vi "TLB Native Dynamic Events ver 0.26d.vi"() -> ()   [LabVIEW 2018] (continued)
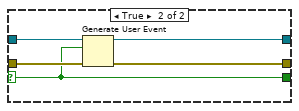
[diagram p2: hidden frame]
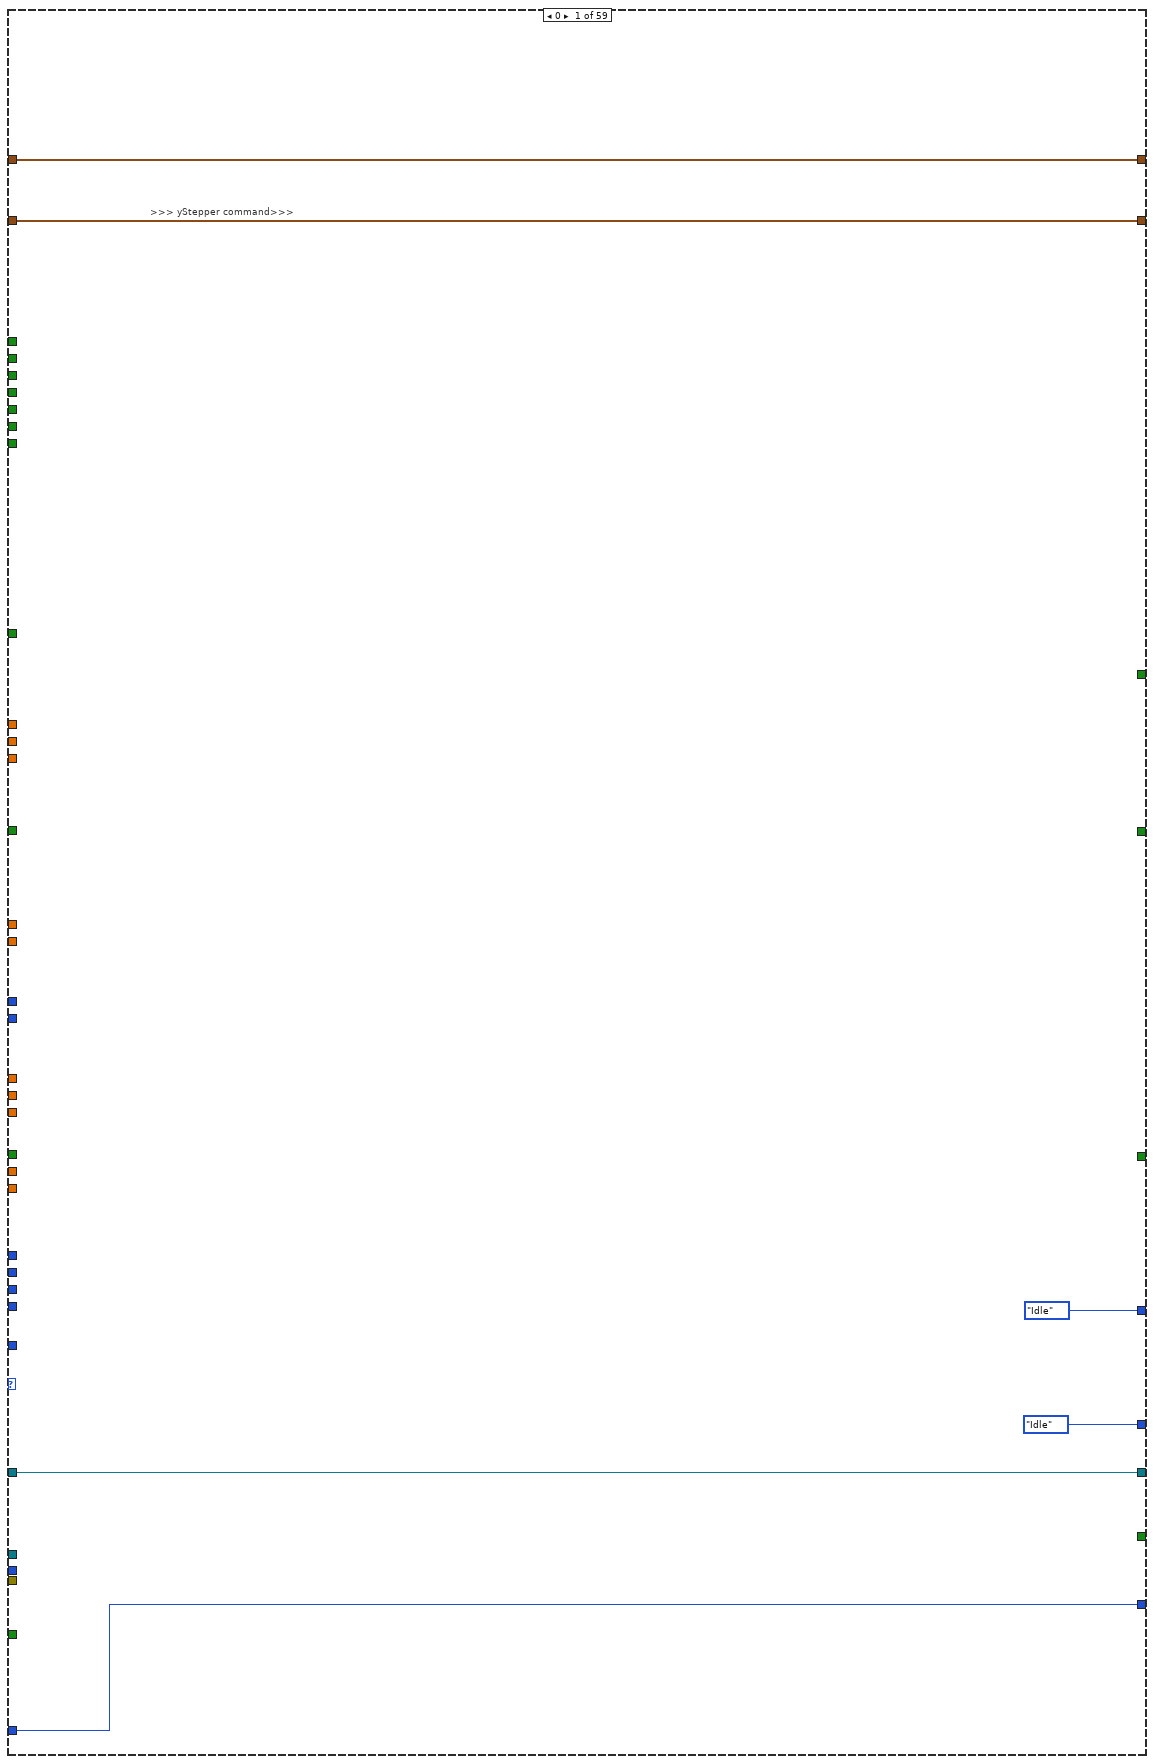
[diagram p5: hidden frame]
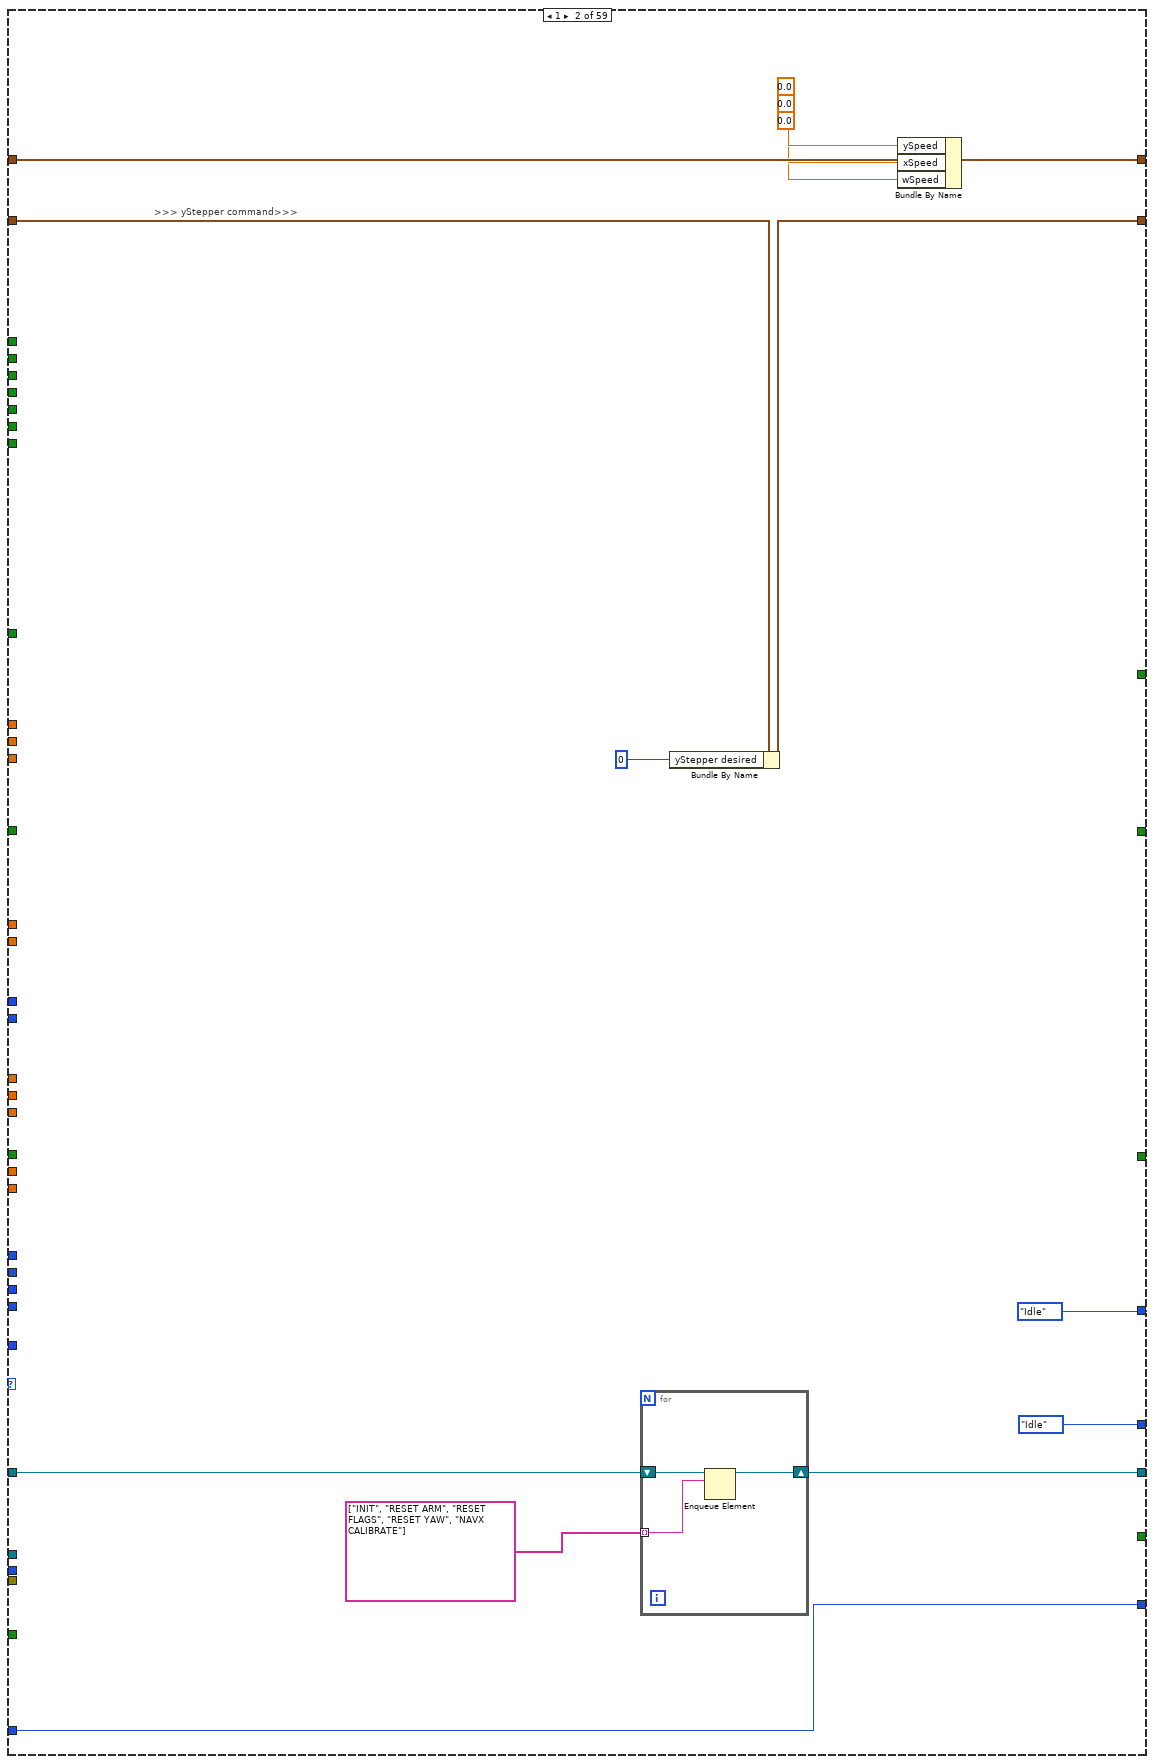
[diagram p6: hidden frame]
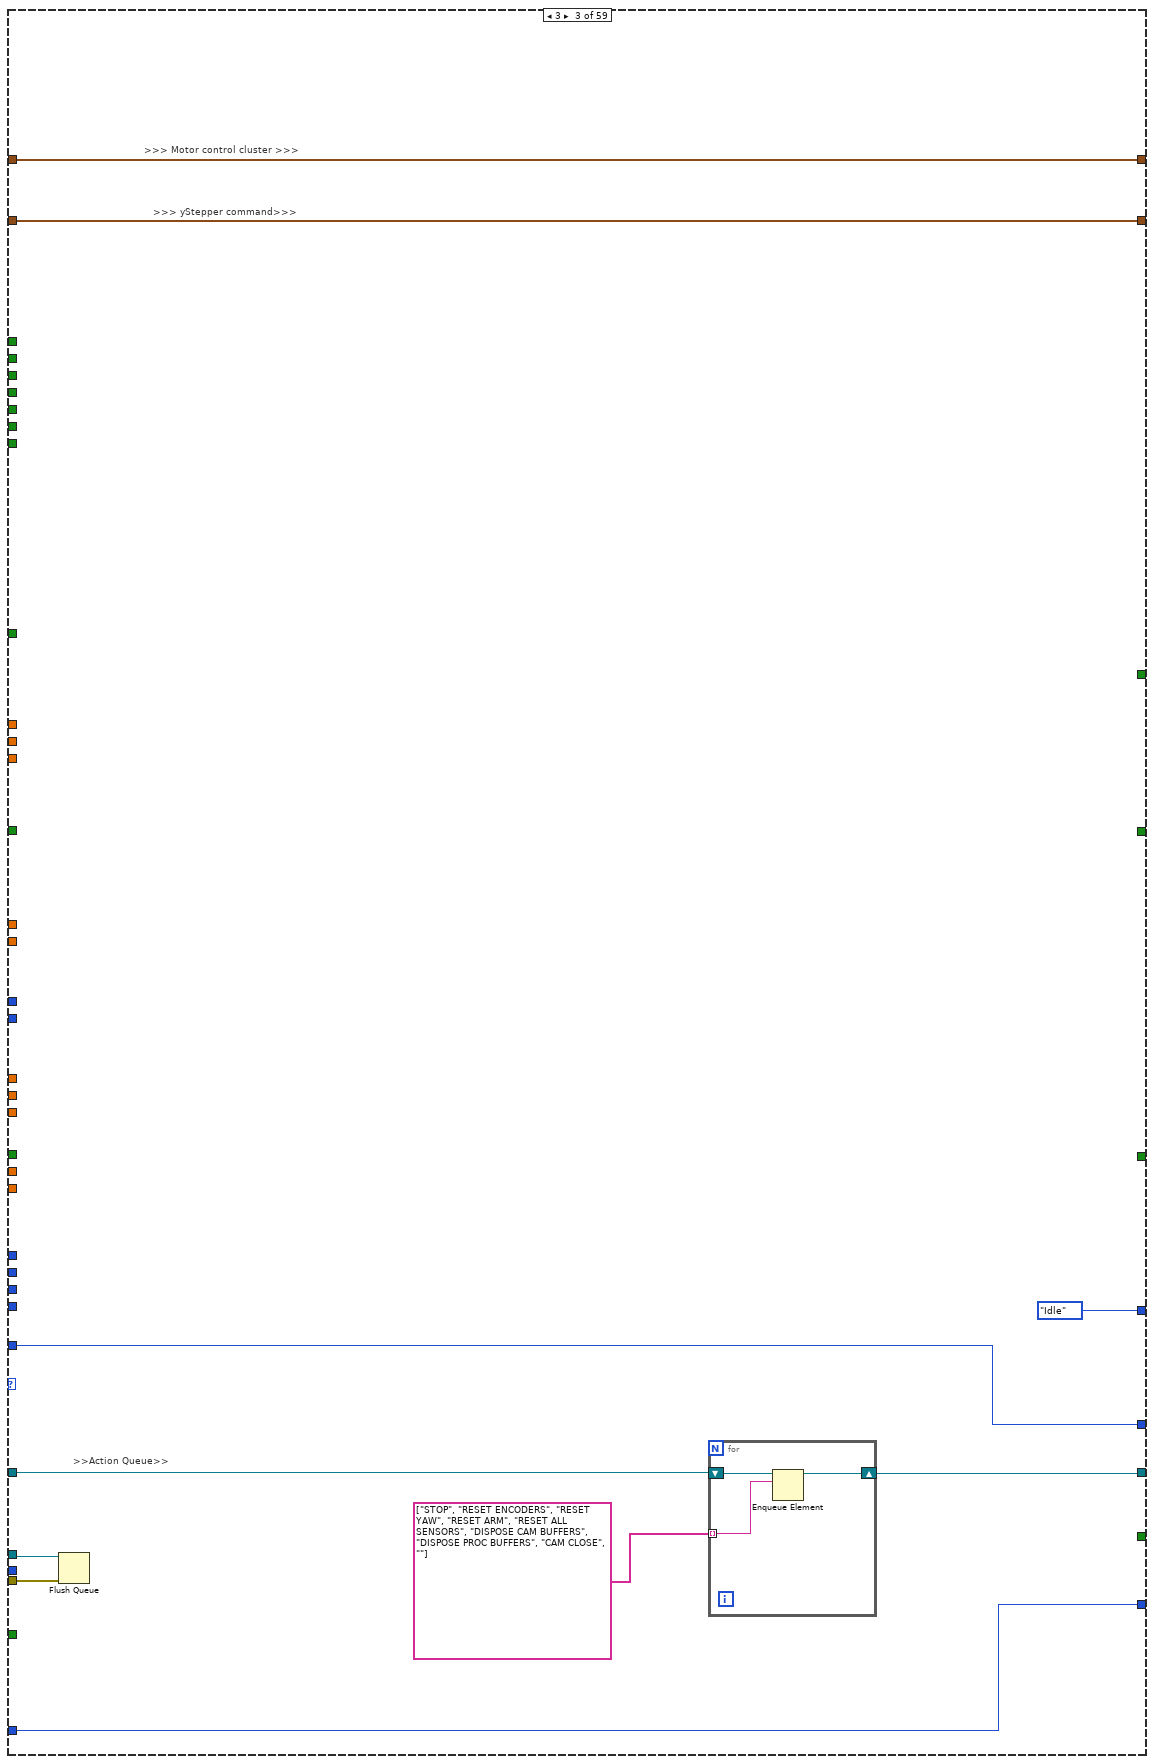
[diagram p7: hidden frame]
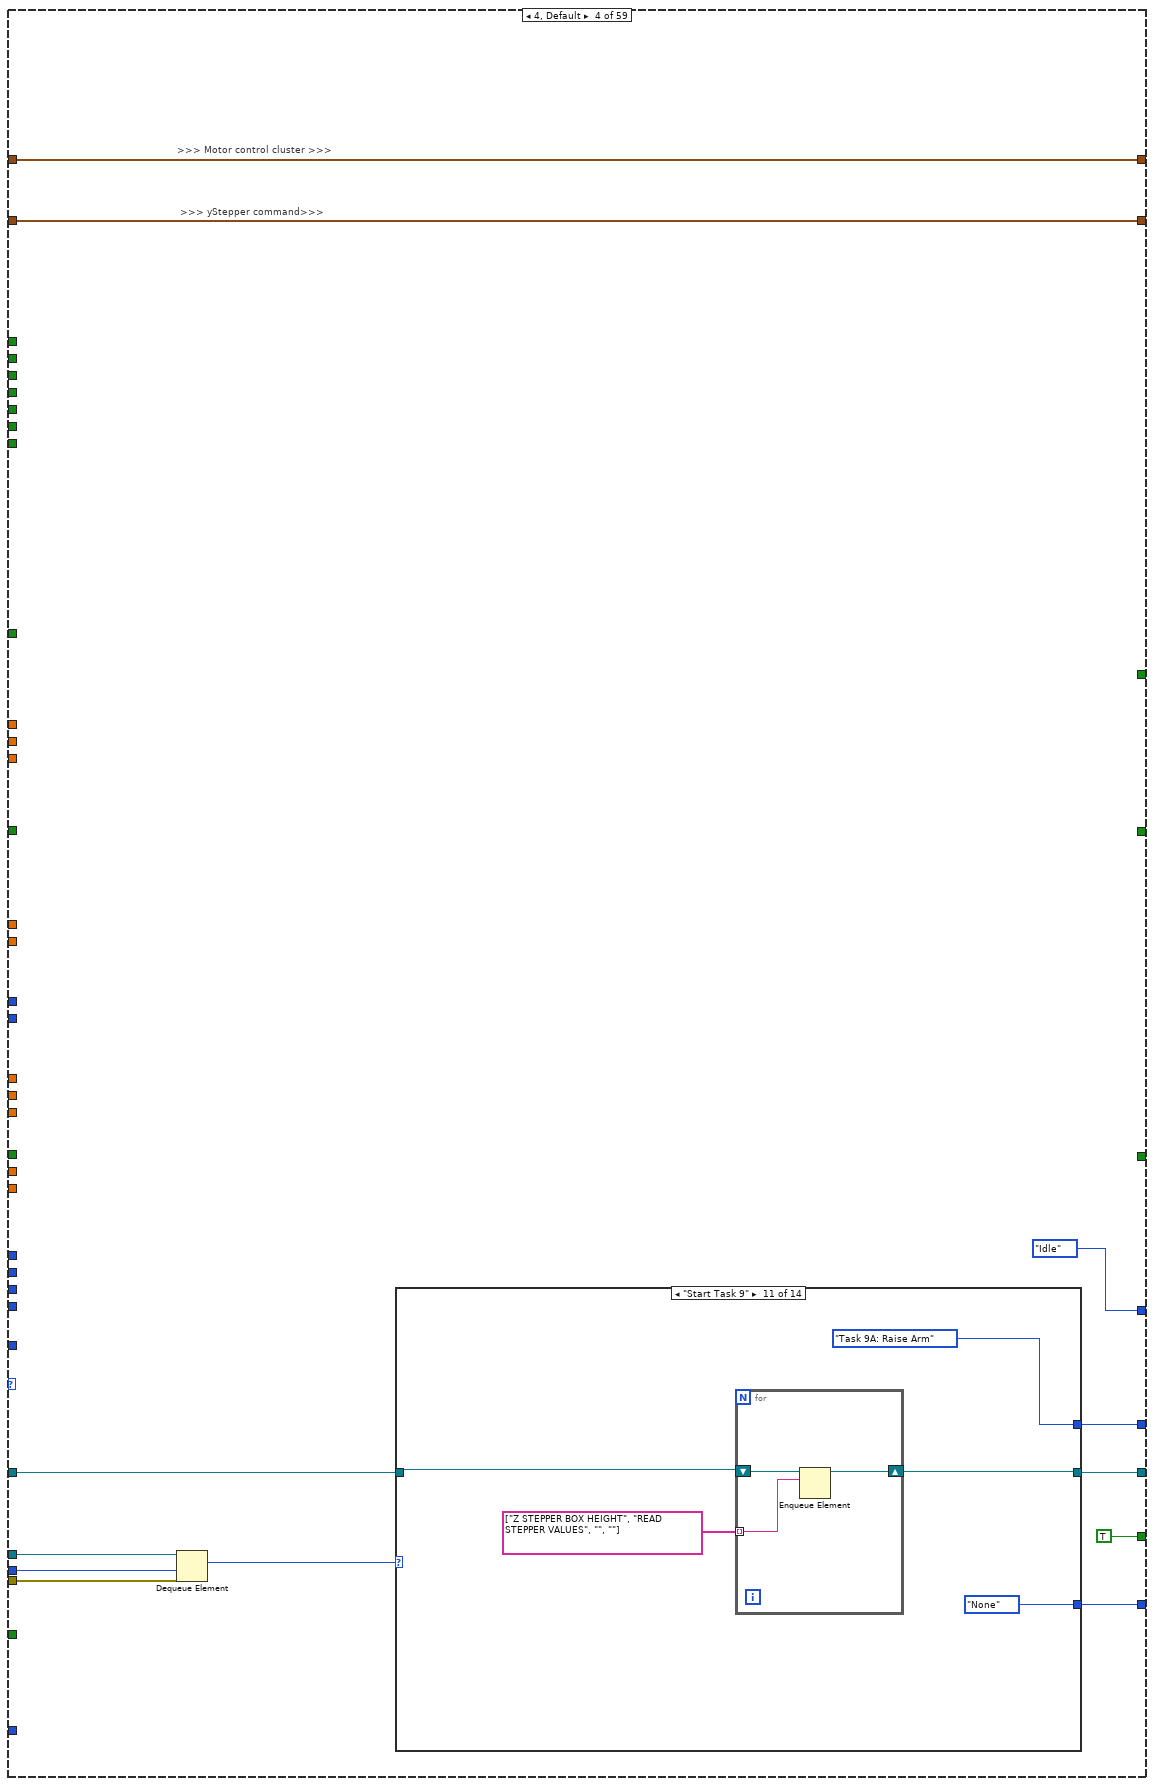
[diagram p8: hidden frame]
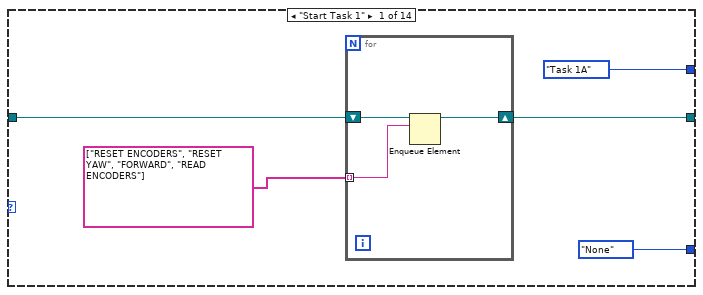
[diagram p9: hidden frame]
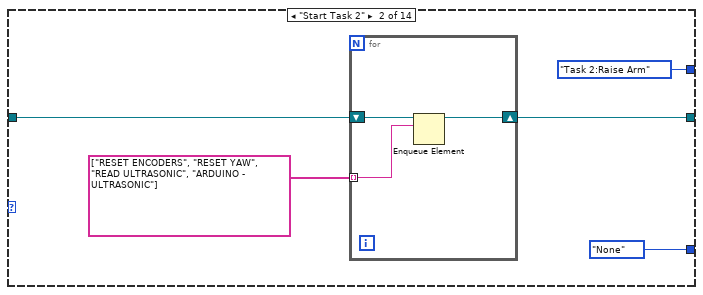
[diagram p10: hidden frame]
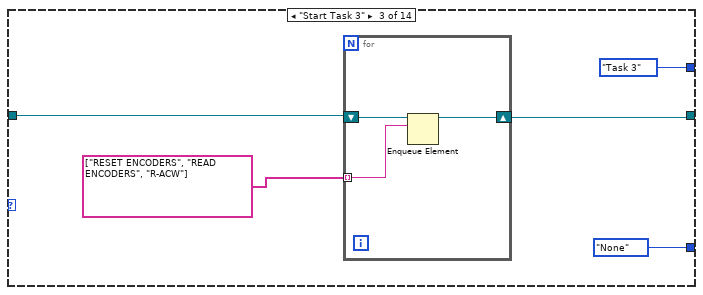
[diagram p11: hidden frame]
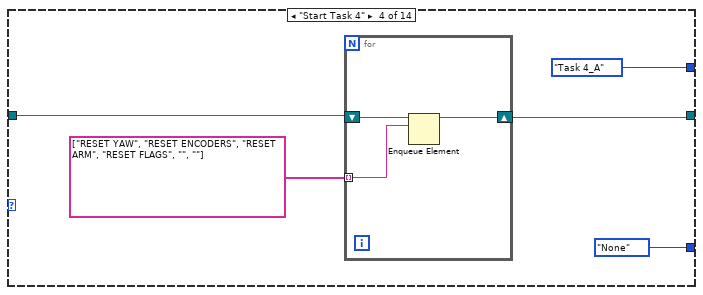
[diagram p12: hidden frame]
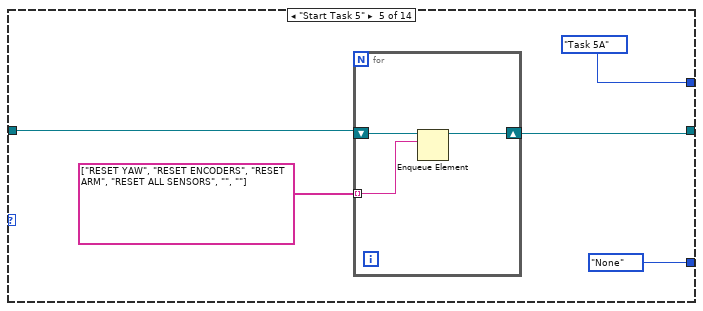
[diagram p13: hidden frame]
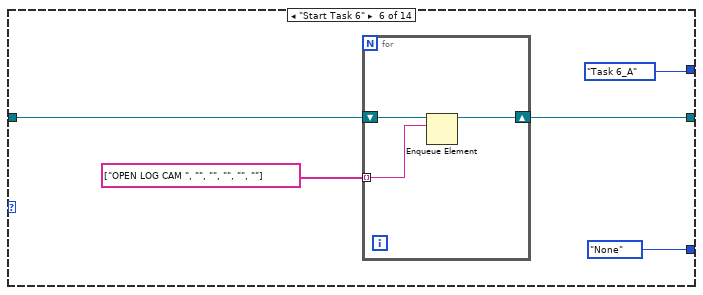
[diagram p14: hidden frame]
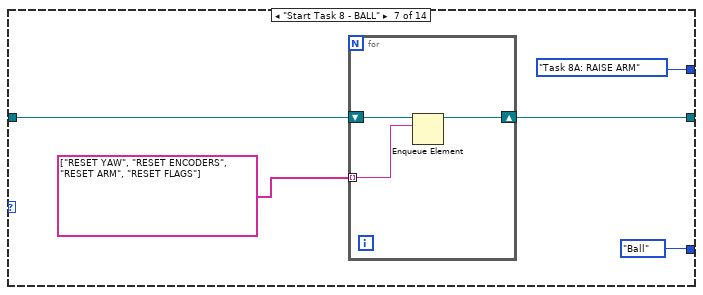
[diagram p15: hidden frame]
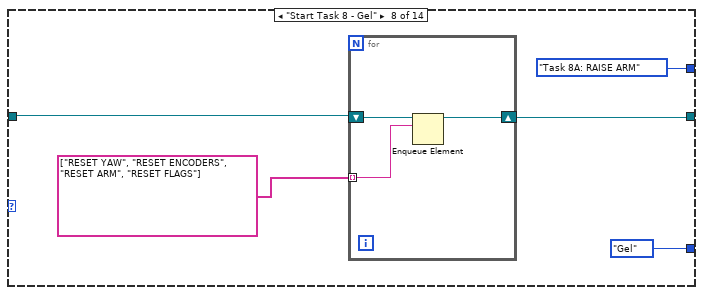
[diagram p16: hidden frame]
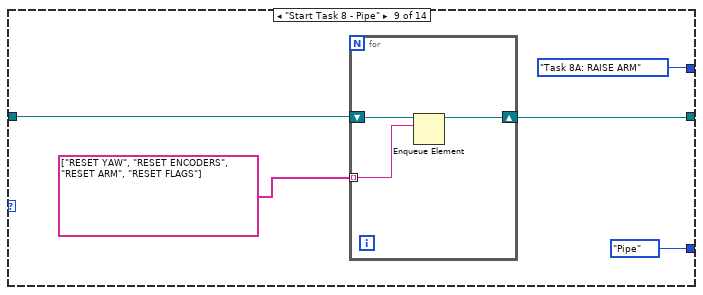
[diagram p17: hidden frame]
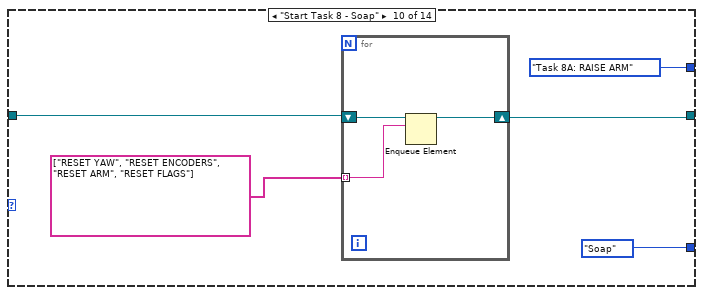
[diagram p18: hidden frame]
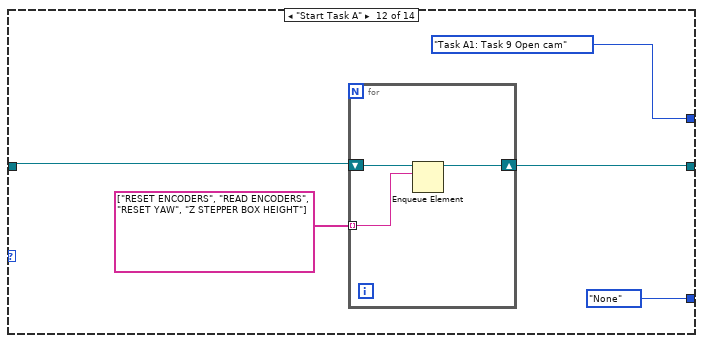
[diagram p19: hidden frame]
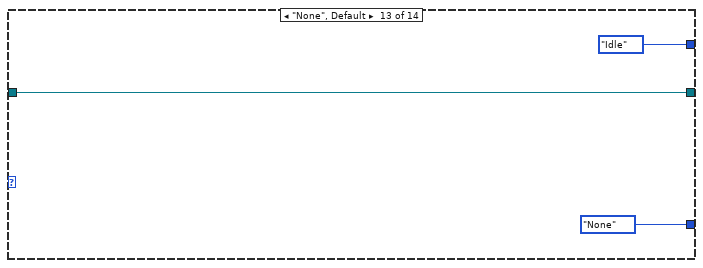
[diagram p20: hidden frame]
                      shift-right: [w2676] -> w2673
                      shift-left: w2674 -> [w2677]
                      tunnel: string[] ["STOP", "RESET ENCODERS", "RESET YAW", "OPEN LIFE CAM", "SET TIMER 2", "RESET FLAGS"] -> [w2675] mode=indexing
                      n870 = Enqueue Element(queue=w2677, element=w2675) -> (queue out=w2676:refnum<queue>)  [unwired: 2 in, 2 out]
                    }
                  }
                }
                n871 = Or(x=w2657, y=w2656) -> (x .or. y?=w2655:bool)
                n872 = Select(t=State_Type_Definitions,_for_0.26g_versions_and_later_2."True Stop" ("Enum"), s=w2656, f=State_Type_Definitions,_for_0.26d_versions_and_later."Task 9Q: SCAN IMAGE" ("Enum")) -> (s? t:f=w2658:u16)
                n873 = Select(t=w2658, s=w2655, f=State_Type_Definitions,_for_0.26d_versions_and_later."Task 9P: MOVE RIGHT" ("Enum")) -> (s? t:f=w2664:u16)
              }
              frame "Exit" {
                n874 = for {
                  shift-right: [w2684] -> w2681
                  shift-left: w2680 -> [w2685]
                  tunnel: string[] ["STOP", "RESET ENCODERS", "RESET YAW", "ARDUINO MODE 0"] -> [w2683] mode=indexing
                  n875 = Enqueue Element(queue=w2685, element=w2683) -> (queue out=w2684:refnum<queue>)  [unwired: 2 in, 2 out]
                }
              }
            }
          }
          frame 54 {
            # ">> Manual override >>"
            n876 = Dequeue Element(queue=w2694, timeout in ms (-1)=w2693, error in (no error)=w2692) -> (element=w2695:T10)  [unwired: 3 out]
            n877 = case shown="\"Start Task 1\", Default" w2695 {
              tunnel: [w2709 State_Type_Definitions,_for_0.26g_versions_and_later_2."True Stop" ("Enum")] -> w2687
              tunnel: [w2707 w2725] -> w2686
              tunnel: w2690 -> [w2706 w2722]
              tunnel: w2691 -> [w2700 _]
              tunnel: [State_Type_Definitions,_for_0.26g_versions_and_later_2."Idle" ("Enum") State_Type_Definitions,_for_0.26g_versions_and_later_2."Shutdown" ("Enum")] -> w2688
              tunnel: w2689 -> [w2699 _]
              frame "Start Task 1", Default {
                # ">> WIill proceed to part ii if not manual override >>"
                # ">>If ENABLE or Trigger is set to true>>"
                n878 = Or(x=w2699, y=w2700) -> (x .or. y?=w2701:bool)
                n879 = case shown="False" w2699 {
                  tunnel: [w2712 w2718] -> w2707
                  tunnel: w2706 -> [w2711 w2717]
                  frame False {
                    n880 = for {
                      shift-right: [w2714] -> w2712
                      shift-left: w2711 -> [w2715]
                      tunnel: string[] ["CAM ACQ", "START TIMER"] ("element") -> [w2713] mode=indexing
                      n881 = Enqueue Element(queue=w2715, element=w2713) -> (queue out=w2714:refnum<queue>)  [unwired: 2 in, 2 out]
                    }
                  }
                  frame True {
                    n882 = for {
                      shift-right: [w2720] -> w2718
                      shift-left: w2717 -> [w2721]
                      tunnel: string[] ["CLOSE CAM", "SET TIMER 5", "", "", "", ""] -> [w2719] mode=indexing
                      n883 = Enqueue Element(queue=w2721, element=w2719) -> (queue out=w2720:refnum<queue>)  [unwired: 2 in, 2 out]
                    }
                  }
                }
                n884 = Select(t=State_Type_Definitions,_for_0.26g_versions_and_later_2."True Stop" ("Enum"), s=w2700, f=State_Type_Definitions,_for_0.26g_versions_and_later_2."Task 9R: PROCESS COLOUR" ("Enum")) -> (s? t:f=w2703:T18)
                n885 = Select(t=w2703, s=w2701, f=State_Type_Definitions,_for_0.26d_versions_and_later."Task 9Q: SCAN IMAGE" ("Enum")) -> (s? t:f=w2709:u16)
              }
              frame "Exit" {
                n886 = for {
                  shift-right: [w2728] -> w2725
                  shift-left: w2722 -> [w2729]
                  tunnel: string[] ["STOP", "RESET ENCODERS", "RESET YAW", ""] -> [w2727] mode=indexing
                  n887 = Enqueue Element(queue=w2729, element=w2727) -> (queue out=w2728:refnum<queue>)  [unwired: 2 in, 2 out]
                }
              }
            }
          }
          frame 55 {
            # ">> Item Selection Bias >>"
            # ">>> Motor control cluster >>>"
            # ">>> yStepper command>>>"
            n888 = Dequeue Element(queue=w2735, timeout in ms (-1)=w2736, error in (no error)=w2737) -> (element=w2739:T10)  [unwired: 3 out]
            n889 = case shown="\"Start Task 1\", Default" w2739 {
              tunnel: w2733 -> [w2745 _]
              tunnel: [w2752 State_Type_Definitions,_for_0.26g_versions_and_later_2."True Stop" ("Enum")] -> w2731
              tunnel: w2738 -> [w2744 _]
              tunnel: w2734 -> [w2751 w2768]
              tunnel: [w2750 w2769] -> w2730
              tunnel: [State_Type_Definitions,_for_0.26g_versions_and_later_2."Idle" ("Enum") State_Type_Definitions,_for_0.26g_versions_and_later_2."Shutdown" ("Enum")] -> w2732
              frame "Start Task 1", Default {
                n890 = case shown="False" w2745 {
                  tunnel: w2751 -> [w2755 w2762]
                  tunnel: [w2756 w2761] -> w2750
                  frame False {
                    n891 = for {
                      tunnel: string[] ["START TIMER", "COLOUR PROCESSING", ""] ("element") -> [w2757] mode=indexing
                      shift-right: [w2759] -> w2756
                      shift-left: w2755 -> [w2758]
                      n892 = Enqueue Element(queue=w2758, element=w2757) -> (queue out=w2759:refnum<queue>)  [unwired: 2 in, 2 out]
                    }
                  }
                  frame True {
                    n893 = for {
                      shift-right: [w2764] -> w2761
                      shift-left: w2762 -> [w2765]
                      tunnel: string[] ["CLOSE CAM", "DISPOSE BUFFERS", "RESET ENCODERS", "RESET YAW", "RESET FLAGS", ""] -> [w2763] mode=indexing
                      n894 = Enqueue Element(queue=w2765, element=w2763) -> (queue out=w2764:refnum<queue>)  [unwired: 2 in, 2 out]
                    }
                  }
                }
                n895 = Or(x=w2745, y=w2744) -> (x .or. y?=w2743:bool)
                n896 = Select(t=State_Type_Definitions,_for_0.26g_versions_and_later_2."True Stop" ("Enum"), s=w2744, f=State_Type_Definitions,_for_0.26g_versions_and_later_2."True Stop" ("Enum")) -> (s? t:f=w2746:T18)
                n897 = Select(t=w2746, s=w2743, f=State_Type_Definitions,_for_0.26g_versions_and_later_2."Task 9R: PROCESS COLOUR" ("Enum")) -> (s? t:f=w2752:T18)
              }
              frame "Exit" {
                n898 = for {
                  shift-right: [w2772] -> w2769
                  shift-left: w2768 -> [w2773]
                  tunnel: string[] ["STOP", "RESET ENCODERS", "RESET YAW", "ARDUINO MODE 0"] -> [w2771] mode=indexing
                  n899 = Enqueue Element(queue=w2773, element=w2771) -> (queue out=w2772:refnum<queue>)  [unwired: 2 in, 2 out]
                }
              }
            }
          }
          frame 56 {
            # ">>> Motor control cluster >>>"
            # ">>> yStepper command>>>"
            # ">> Manual override >>"
            n900 = Dequeue Element(queue=w2785, timeout in ms (-1)=w2781, error in (no error)=w2784) -> (element=w2786:T10)  [unwired: 3 out]
            n901 = case shown="\"Start Task 1\", Default" w2786 {
              tunnel: [w2797 State_Type_Definitions,_for_0.26g_versions_and_later_2."True Stop" ("Enum")] -> w2779
              tunnel: [w2795 w2812] -> w2778
              tunnel: w2782 -> [w2794 _]
              tunnel: w2783 -> [w2788 _]
              tunnel: [State_Type_Definitions,_for_0.26g_versions_and_later_2."Idle" ("Enum") State_Type_Definitions,_for_0.26g_versions_and_later_2."Shutdown" ("Enum")] -> w2780
              tunnel: w2774 -> [w2787 _]
              frame "Start Task 1", Default {
                # ">> WIill proceed to part ii if not manual override >>"
                # ">>If ENABLE or Trigger is set to true>>"
                n902 = Or(x=w2787, y=w2788) -> (x .or. y?=w2789:bool)
                n903 = case shown="False" w2787 {
                  tunnel: [w2800 w2806] -> w2795
                  tunnel: w2794 -> [w2799 w2805]
                  frame False {
                    n904 = for {
                      shift-right: [w2802] -> w2800
                      shift-left: w2799 -> [w2803]
                      tunnel: string[] ["Task 9", ""] ("element") -> [w2801] mode=indexing
                      n905 = Enqueue Element(queue=w2803, element=w2801) -> (queue out=w2802:refnum<queue>)  [unwired: 2 in, 2 out]
                    }
                  }
                  frame True {
                    n906 = for {
                      shift-right: [w2808] -> w2806
                      shift-left: w2805 -> [w2809]
                      tunnel: string[] ["ARDUINO - ULTRASONIC", "READ NAVX", "RESET FLAGS", "", "", ""] -> [w2807] mode=indexing
                      n907 = Enqueue Element(queue=w2809, element=w2807) -> (queue out=w2808:refnum<queue>)  [unwired: 2 in, 2 out]
                    }
                  }
                }
                n908 = Select(t=State_Type_Definitions,_for_0.26g_versions_and_later_2."True Stop" ("Enum"), s=w2788, f=State_Type_Definitions,_for_0.26g_versions_and_later_2."True Stop" ("Enum")) -> (s? t:f=w2791:T18)
                n909 = Select(t=w2791, s=w2789, f=State_Type_Definitions,_for_0.26g_versions_and_later_2."Task A1: Task 9 Open cam" ("Enum")) -> (s? t:f=w2797:T18)
              }
              frame "Exit" {
                n910 = for {
                  shift-right: [w2815] -> w2812
                  shift-left: _ -> [w2816]
                  tunnel: string[] ["STOP", "RESET ENCODERS", "RESET YAW", ""] -> [w2814] mode=indexing
                  n911 = Enqueue Element(queue=w2816, element=w2814) -> (queue out=w2815:refnum<queue>)  [unwired: 2 in, 2 out]
                }
              }
            }
          }
          frame 57 {
            # ">>> Motor control cluster >>>"
            # ">>> yStepper command>>>"
            n912 = Dequeue Element(queue=w2830, timeout in ms (-1)=w2829, error in (no error)=w2828) -> (element=w2832:T10)  [unwired: 3 out]
            n913 = In Range and Coerce(upper limit=65.0, x=w2822, lower limit=58.0) -> (In Range?=w2819:bool)  [unwired: 1 out]
            n914 = case shown="\"Start Task 1\", Default" w2832 {
              tunnel: w2823 -> [w2835 _]
              tunnel: [w2843 State_Type_Definitions,_for_0.26g_versions_and_later_2."True Stop" ("Enum")] -> w2825
              tunnel: w2831 -> [w2841 w2859]
              tunnel: [w2840 w2858] -> w2824
              tunnel: [State_Type_Definitions,_for_0.26g_versions_and_later_2."Idle" ("Enum") State_Type_Definitions,_for_0.26g_versions_and_later_2."Shutdown" ("Enum")] -> w2826
              tunnel: w2819 -> [w2833 _]
              frame "Start Task 1", Default {
                n915 = Or(x=w2833, y=w2835) -> (x .or. y?=w2834:bool)
                n916 = case shown="True" w2833 {
                  tunnel: w2841 -> [w2846 w2852]
                  tunnel: [w2845 w2850] -> w2840
                  frame False {
                    n917 = for {
                      shift-right: [w2848] -> w2845
                      shift-left: w2846 -> [w2849]
                      tunnel: string[] ["READ NAVX", "R-CW", "READ ULTRASONIC"] ("element") -> [w2847] mode=indexing
                      n918 = Enqueue Element(queue=w2849, element=w2847) -> (queue out=w2848:refnum<queue>)  [unwired: 2 in, 2 out]
                    }
                  }
                  frame True {
                    n919 = for {
                      shift-right: [w2854] -> w2850
                      shift-left: w2852 -> [w2855]
                      tunnel: string[] ["STOP", "RESET ENCODERS", "RESET YAW", "READ IR", "ARDUINO - ULTRASONIC"] -> [w2853] mode=indexing
                      n920 = Enqueue Element(queue=w2855, element=w2853) -> (queue out=w2854:refnum<queue>)  [unwired: 2 in, 2 out]
                    }
                  }
                }
                n921 = Select(t=State_Type_Definitions,_for_0.26g_versions_and_later_2."True Stop" ("Enum"), s=w2835, f=State_Type_Definitions,_for_0.26g_versions_and_later_2."Task A3: Task 9 Set Timer") -> (s? t:f=w2837:T18)
                n922 = Select(t=w2837, s=w2834, f=State_Type_Definitions,_for_0.26g_versions_and_later_2."Task A2: Task 9 Move Arm" ("Enum")) -> (s? t:f=w2843:T18)
              }
              frame "Exit" {
                n923 = for {
                  shift-right: [w2862] -> w2858
                  shift-left: w2859 -> [w2863]
                  tunnel: string[] ["STOP", "RESET ENCODERS", "RESET YAW", ""] -> [w2861] mode=indexing
                  n924 = Enqueue Element(queue=w2863, element=w2861) -> (queue out=w2862:refnum<queue>)  [unwired: 2 in, 2 out]
                }
              }
            }
          }
          frame 58 {
            (unwired) 50.0 ("y")
            (unwired) 15.0 ("y")
            # ">> Item Selection Bias >>"
            # ">> Wall detected >>"
            # ">> Manual override >>"
            # ">>> Motor control cluster >>>"
            # ">>Table or wall detectected>>"
            # ">>Action Queue>>"
            # ">>> yStepper command>>>"
            n925 = Dequeue Element(queue=w2879, timeout in ms (-1)=w2878, error in (no error)=w2877) -> (element=w2880:T10)  [unwired: 3 out]
            n926 = Less?(x=w2866, y=100.0) -> (x < y?=w2867:bool)
            n927 = Not Equal To 0?(x=w2866) -> (x != 0?=w2865:bool)
            n928 = And(x=w2865, y=w2867) -> (x .and. y?=w2864:bool)
            n929 = case shown="\"Start Task 1\", Default" w2880 {
              tunnel: w2875 -> [w2881 _]
              tunnel: [w2891 State_Type_Definitions,_for_0.26g_versions_and_later_2."True Stop" ("Enum")] -> w2872
              tunnel: w2876 -> [w2889 w2907]
              tunnel: [w2888 w2906] -> w2871
              tunnel: [State_Type_Definitions,_for_0.26g_versions_and_later_2."Idle" ("Enum") State_Type_Definitions,_for_0.26g_versions_and_later_2."Shutdown" ("Enum")] -> w2874
              tunnel: w2864 -> [w2882 _]
              frame "Start Task 1", Default {
                n930 = Or(x=w2881, y=w2882) -> (x .or. y?=w2883:bool)
                n931 = case shown="False" w2882 {
                  tunnel: w2889 -> [w2894 w2900]
                  tunnel: [w2893 w2898] -> w2888
                  frame False {
                    n932 = for {
                      shift-right: [w2896] -> w2893
                      shift-left: w2894 -> [w2897]
                      tunnel: string[] ["READ IR", "FORWARD - IR ASSIST", "READ ULTRASONIC"] ("element") -> [w2895] mode=indexing
                      n933 = Enqueue Element(queue=w2897, element=w2895) -> (queue out=w2896:refnum<queue>)  [unwired: 2 in, 2 out]
                    }
                  }
                  frame True {
                    n934 = for {
                      shift-right: [w2902] -> w2898
                      shift-left: w2900 -> [w2903]
                      tunnel: string[] ["STOP", "RESET ENCODERS", "RESET YAW", ""] -> [w2901] mode=indexing
                      n935 = Enqueue Element(queue=w2903, element=w2901) -> (queue out=w2902:refnum<queue>)  [unwired: 2 in, 2 out]
                    }
                  }
                }
                n936 = Select(t=State_Type_Definitions,_for_0.26g_versions_and_later_2."True Stop" ("Enum"), s=w2881, f=State_Type_Definitions,_for_0.26g_versions_and_later_2."Task A4: Tasl 9 Capture images") -> (s? t:f=w2885:T18)
                n937 = Select(t=w2885, s=w2883, f=State_Type_Definitions,_for_0.26g_versions_and_later_2."Task A3: Task 9 Set Timer" ("Enum")) -> (s? t:f=w2891:T18)
              }
              frame "Exit" {
                n938 = for {
                  shift-right: [w2910] -> w2906
                  shift-left: w2907 -> [w2911]
                  tunnel: string[] ["STOP", "RESET ENCODERS", "RESET YAW", ""] -> [w2909] mode=indexing
                  n939 = Enqueue Element(queue=w2911, element=w2909) -> (queue out=w2910:refnum<queue>)  [unwired: 2 in, 2 out]
                }
              }
            }
          }
          frame 59 {
            # ">>> Motor control cluster >>>"
            # ">>> yStepper command>>>"
            # ">> Item Selection Bias >>"
            n940 = Less?(x=w2915, y=-40.0) -> (x < y?=w2913:bool)
            n941 = Dequeue Element(queue=w2921, timeout in ms (-1)=w2920, error in (no error)=w2919) -> (element=w2923:T10)  [unwired: 3 out]
            n942 = case shown="\"Start Task 1\", Default" w2923 {
              tunnel: w2913 -> [w2929 _]
              tunnel: [w2936 State_Type_Definitions,_for_0.26g_versions_and_later_2."True Stop" ("Enum")] -> w2917
              tunnel: w2918 -> [w2928 _]
              tunnel: w2922 -> [w2935 w2952]
              tunnel: [w2934 w2953] -> w2912
              tunnel: [State_Type_Definitions,_for_0.26g_versions_and_later_2."Idle" ("Enum") State_Type_Definitions,_for_0.26g_versions_and_later_2."Shutdown" ("Enum")] -> w2916
              frame "Start Task 1", Default {
                n943 = case shown="True" w2929 {
                  tunnel: w2935 -> [w2939 w2946]
                  tunnel: [w2940 w2945] -> w2934
                  frame False {
                    n944 = for {
                      tunnel: string[] ["READ ENCODERS", "R-CW"] ("element") -> [w2941] mode=indexing
                      shift-right: [w2943] -> w2940
                      shift-left: w2939 -> [w2942]
                      n945 = Enqueue Element(queue=w2942, element=w2941) -> (queue out=w2943:refnum<queue>)  [unwired: 2 in, 2 out]
                    }
                  }
                  frame True {
                    n946 = for {
                      shift-right: [w2948] -> w2945
                      shift-left: w2946 -> [w2949]
                      tunnel: string[] ["STOP", "RESET ENCODERS", "RESET FLAGS", "RESET YAW", "READ IR", ""] -> [w2947] mode=indexing
                      n947 = Enqueue Element(queue=w2949, element=w2947) -> (queue out=w2948:refnum<queue>)  [unwired: 2 in, 2 out]
                    }
                  }
                }
                n948 = Or(x=w2929, y=w2928) -> (x .or. y?=w2927:bool)
                n949 = Select(t=State_Type_Definitions,_for_0.26g_versions_and_later_2."True Stop" ("Enum"), s=w2928, f=State_Type_Definitions,_for_0.26g_versions_and_later_2."Task A3: Task 9 Set Timer" ("Enum")) -> (s? t:f=w2930:T18)
                n950 = Select(t=w2930, s=w2927, f=State_Type_Definitions,_for_0.26g_versions_and_later_2."Task A4: Tasl 9 Capture images" ("Enum")) -> (s? t:f=w2936:T18)
              }
              frame "Exit" {
                n951 = for {
                  shift-right: [w2956] -> w2953
                  shift-left: w2952 -> [w2957]
                  tunnel: string[] ["STOP", "RESET ENCODERS", "RESET YAW", "ARDUINO MODE 0"] -> [w2955] mode=indexing
                  n952 = Enqueue Element(queue=w2957, element=w2955) -> (queue out=w2956:refnum<queue>)  [unwired: 2 in, 2 out]
                }
              }
            }
          }
        }
        "Object Detection" <- w320
        "Ultrasonic sensors" <- w343
        "Encoder values" <- w332
        "Stepper position values" <- w316
        "NAVX Values" <- w314
        "IR Sensors" <- w306
        "Line sensors" <- w301
        "Time cluster" <- w312
        "Box Colour Detection" <- w294
      }
    }
    "Object recognition mode" <- w220
    "Front Ultrasonic obstruct" <- w217
    "Front IR obstruct" <- w216
    "Table IR obstruct" <- w215
    n953 = local write "Green LED"(w230) -> ()
  }
  n954 = while {
    stop <- w3857 stop-if-true
    n955 = call "MOTOR CONTROL WITH PID AE.vi"("AE Mode"=MOTOR_CONTROL_WITH_PID_AE_DATA_MODE_TYPE_DEF."Read from AE") -> ("Speed & distance"=→"Speed & distance":T15)  [unwired: 3 in]
    n956 = call "FGV Stop.vi"("Init/Read/Write State"=States_for_Action_Engine."Read") -> ("Output node"=w3857:bool)  [unwired: 2 in, 1 out]
    n957 = Wait (ms)(milliseconds to wait=u32 5) -> ()  [unwired: 1 out]
  }
  n958 = call <vilib>:"DIO Close.vi"("error in (no error)"=w23, "DIO Info In"=w26) -> ()  [unwired: 9 in, 1 out]
  n959 = call <vilib>:"DIO Close.vi"("error in (no error)"=w33, "DIO Info In"=w35) -> ()  [unwired: 9 in, 1 out]
  n960 = call <vilib>:"NavX Close.vi"("error in (no error)"=w10, "NavX Info In"=w9) -> ()  [unwired: 9 in, 1 out]
  n961 = call <vilib>:"DIO Close.vi"("error in (no error)"=w28, "DIO Info In"=w30) -> ()  [unwired: 9 in, 1 out]
  n962 = call <vilib>:"DIO Close.vi"("error in (no error)"=w17, "DIO Info In"=w18) -> ()  [unwired: 9 in, 1 out]
  n963 = call <vilib>:"DIO Close.vi"("error in (no error)"=w12, "DIO Info In"=w13) -> ()  [unwired: 9 in, 1 out]
  n964 = Merge Errors "Merge Errors"(w63, w62) -> (w45:errorcluster)
  n965 = Merge Errors(w49, w45) -> (w44:errorcluster)
  n966 = Destroy User Event(user event=w67, error in=w44) -> ()  [unwired: 1 out]
  n967 = Release Queue(queue=w40, error in (no error)=w44) -> (error out=→"Queue Errors":errorcluster)  [unwired: 1 in, 2 out]
  n968 = Release Queue(queue=w57, error in (no error)=w44) -> ()  [unwired: 1 in, 3 out]
  n969 = Destroy User Event(user event=w66, error in=w44) -> ()  [unwired: 1 out]
  n970 = Unregister For Events(event registration refnum=w58, error in=w44) -> ()  [unwired: 1 out]
